vi "UHR-Fleezers Control (host) - 10.0.vi"() -> ()   [LabVIEW 2009] (continued)
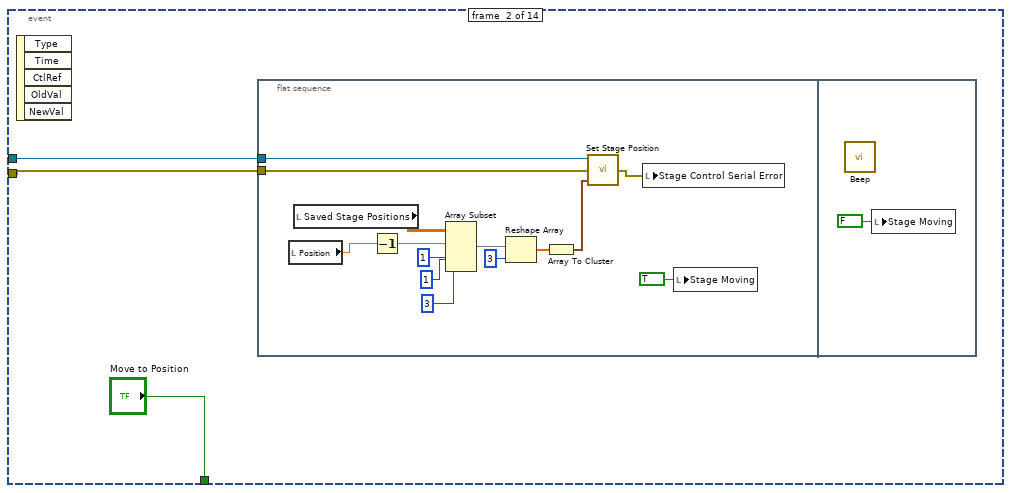
[diagram p2: hidden frame]
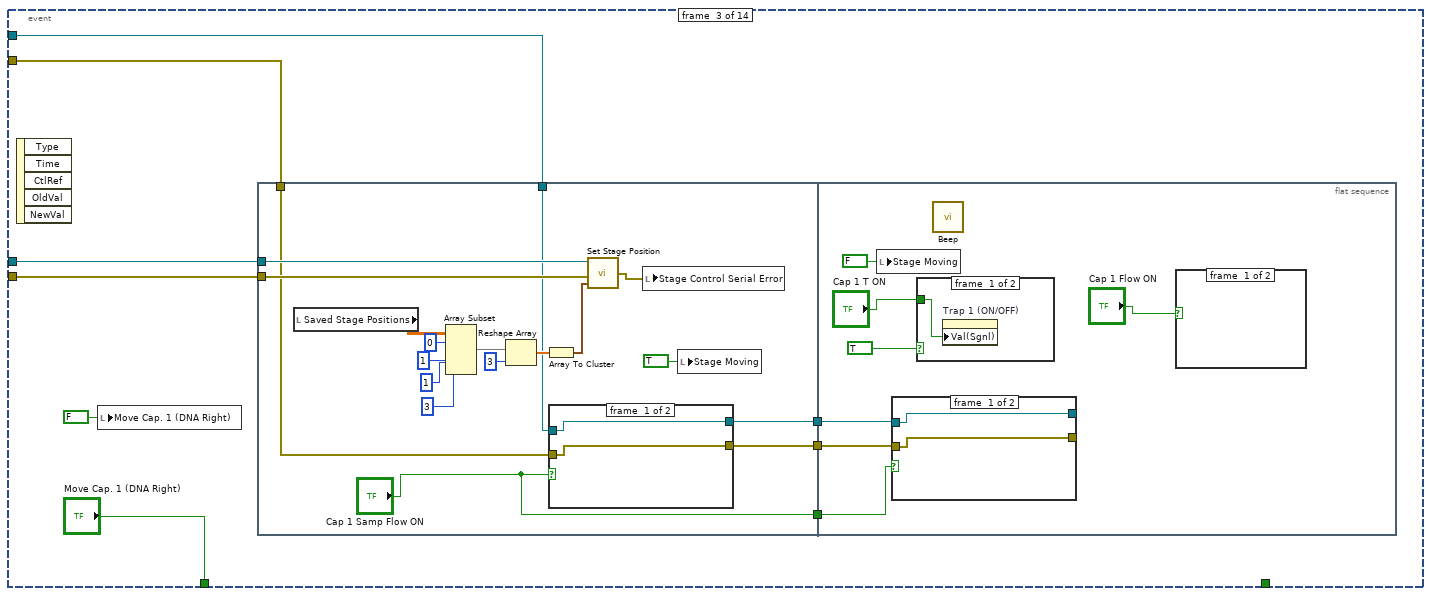
[diagram p3: hidden frame]
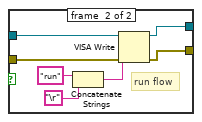
[diagram p4: hidden frame]
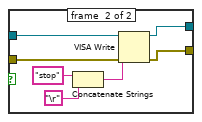
[diagram p5: hidden frame]
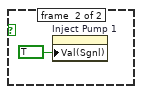
[diagram p6: hidden frame]
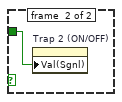
[diagram p7: hidden frame]
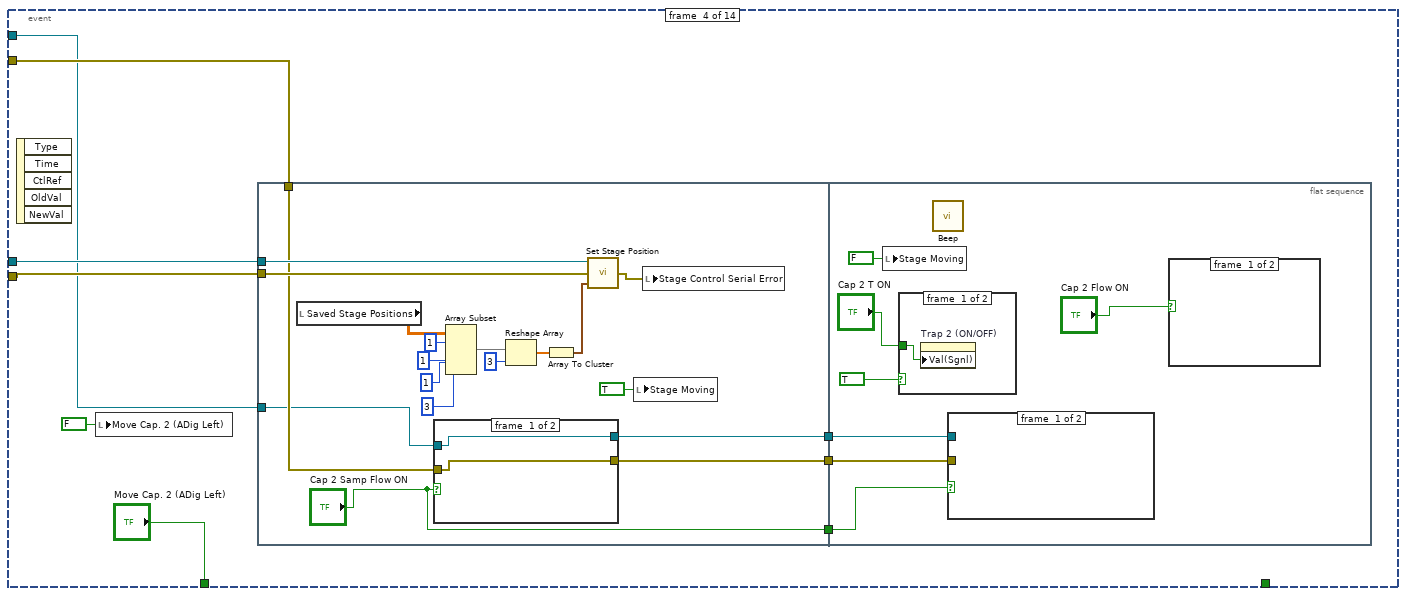
[diagram p8: hidden frame]
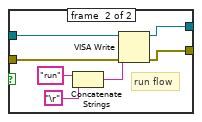
[diagram p9: hidden frame]
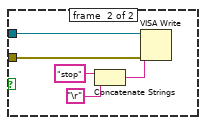
[diagram p10: hidden frame]
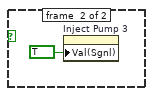
[diagram p11: hidden frame]
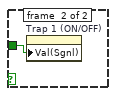
[diagram p12: hidden frame]
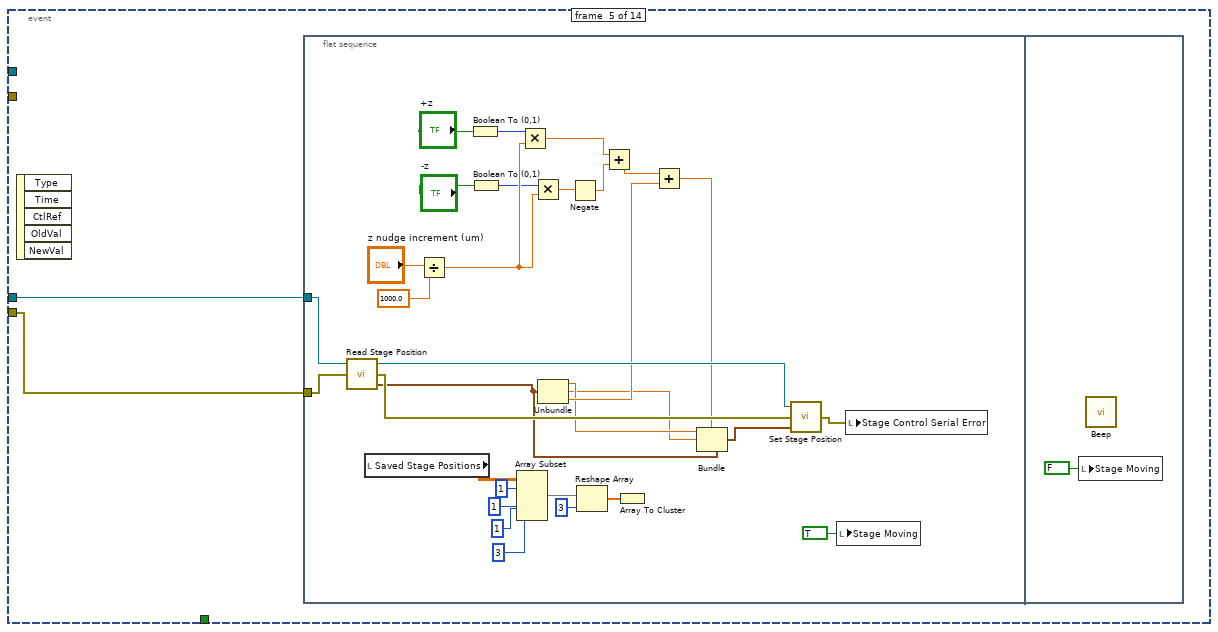
[diagram p13: hidden frame]
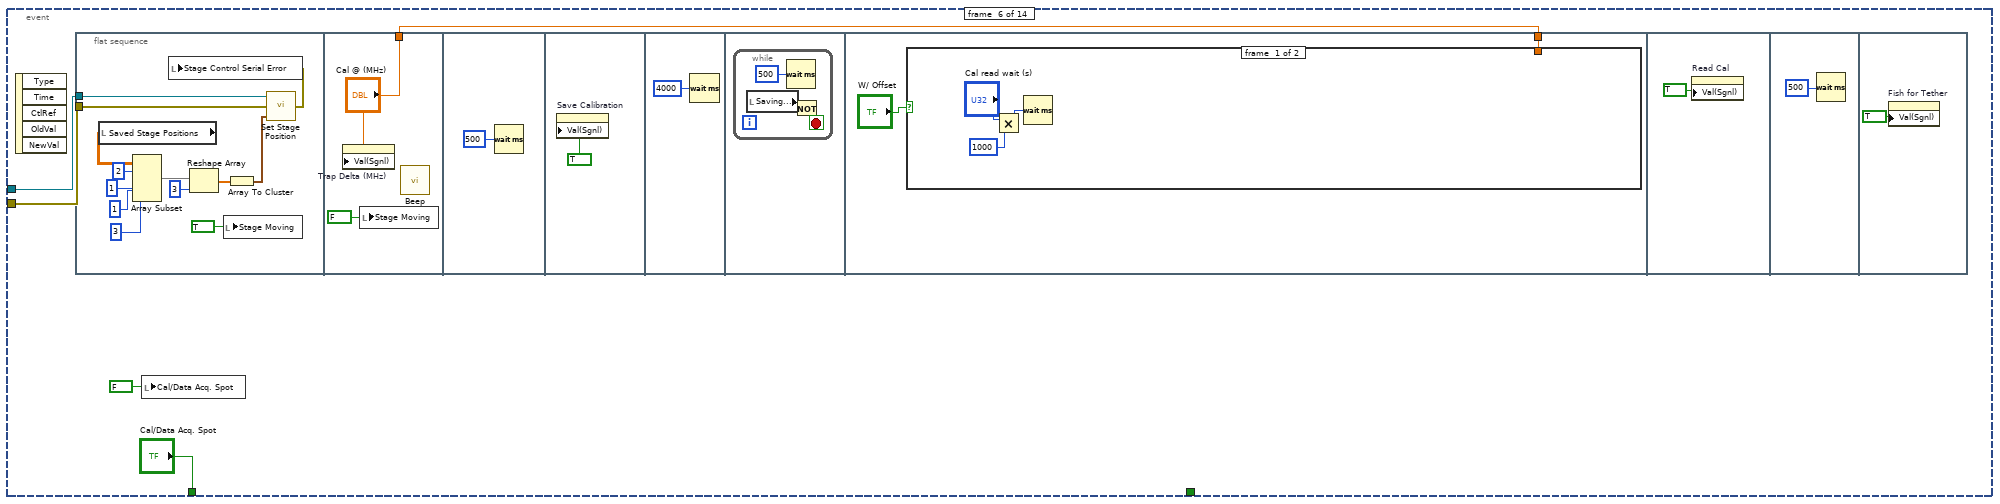
[diagram p14: hidden frame]
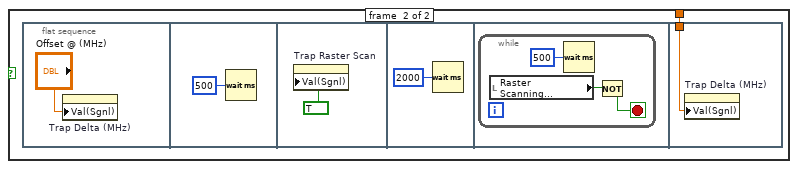
[diagram p15: hidden frame]
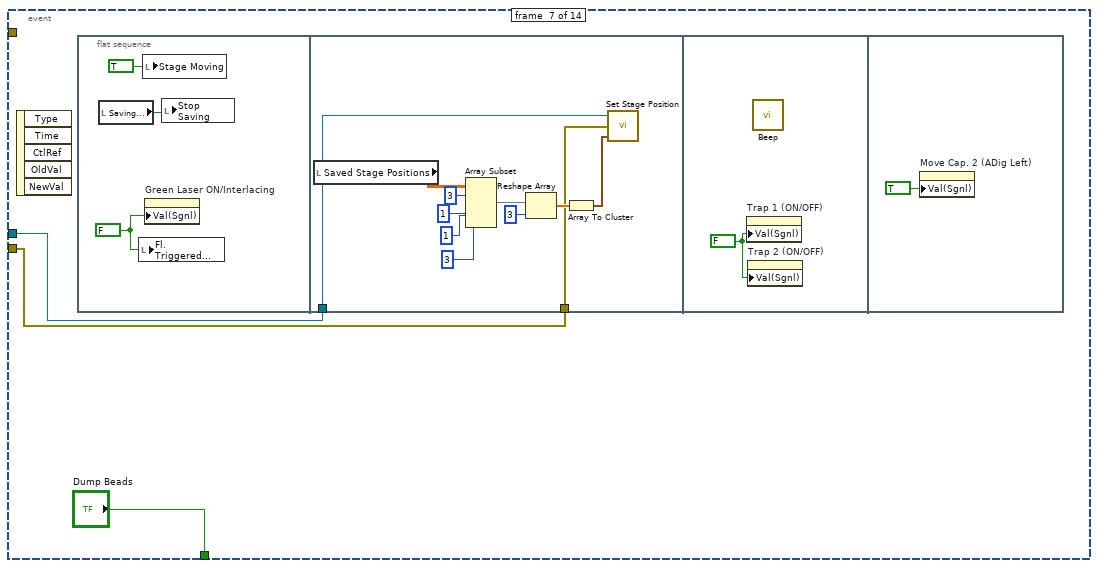
[diagram p16: hidden frame]
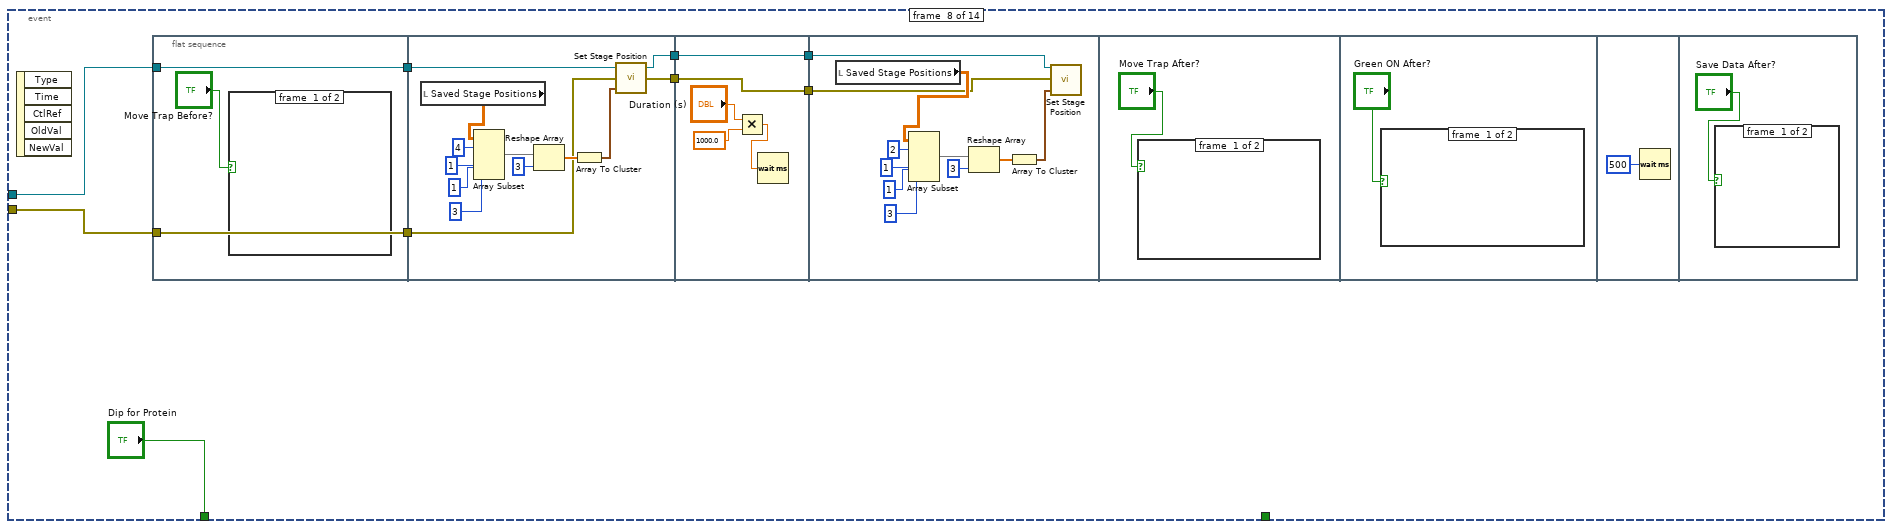
[diagram p17: hidden frame]
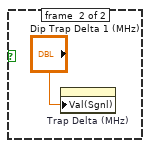
[diagram p18: hidden frame]
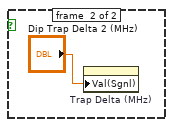
[diagram p19: hidden frame]
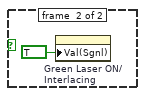
[diagram p20: hidden frame]
                          n1924 = local write "BD 2 Frequency 1 (MHz)"(w8168) -> ()
                          n1925 = local write "BD 1 Frequency 1 (MHz)"(w8170) -> ()
                        }
                      }
                    }
                    frame #1 {
                    }
                  }
                }
                event #1 {
                  n1926 = event-data() -> ("Button"=w8173:u16)  [unwired: 8 out]
                  n1927 = case shown="3" w8173 {
                    tunnel: [FALSE TRUE] -> w8174
                    frame #0 {
                    }
                    frame #1 {
                      n1928 = local write "Manipulating Trap"(FALSE ("Manipulating Trap")) -> ()
                    }
                  }
                }
              }
            }
          }
        }
      }
      event #1 {
        n1929 = event-data() -> ()  [unwired: 6 out]
      }
    }
    n1930 = local read "Stop All"() -> (w7995:bool)
    n1931 = node-c288() -> ()  [unwired: 2 out]
  }
  n1932 = timed-loop "Run Scripts, including: stage motion" {
    tunnel: w44 -> [w8180]
    tunnel: w43 -> [w8181]
    tunnel: [w8181] -> w42
    tunnel: [w8180] -> w41
    timing: w39 -> [_]
    timing-out: [_] -> w38
    tunnel: w22 -> [w8179]
    tunnel: w23 -> [w8178]
    stop <- w8182 stop-if-true
    n1933 = node-c288() -> ()  [unwired: 1 in, 1 out]
    n1934 = event shown="[10] \"Got ADig bead\": Value Change" {
      selector: _ -> [_ _ _ _ _ _ _ _ _ _ _ _ _ _]
      dyn-events: _ -> [_ _ _ _ _ _ _ _ _ _ _ _ _ _]
      timeout: _ -> [_ _ _ _ _ _ _ _ _ _ _ _ _ _]
      tunnel: ["Set Position" "Move to Position" "Move Cap. 1 (DNA Right)" "Move Cap. 2 (ADig Left)" _ "Cal/Data Acq. Spot" "Dump Beads" "Dip for Protein" _ _ "Got ADig bead" "Got DNA bead" "Take Detection Laser\nImage" _] -> _
      tunnel: [_ _ _ _ _ _ _ _ _ _ _ _ _ w8600] -> w8182
      tunnel: w8180 -> [w8200 w8208 w8232 w8287 w8332 w8368 w8409 w8434 w8484 w8510 _ _ _ _]
      tunnel: w8181 -> [w8201 w8209 w8233 w8288 w8333 w8369 w8410 w8435 w8485 w8511 _ _ _ _]
      tunnel: w8179 -> [_ _ w8230 w8284 _ _ _ _ _ _ _ _ _ _]
      tunnel: w8178 -> [_ _ w8229 w8285 _ _ _ _ _ _ _ _ _ _]
      event #0 {
        n1935 = event-data() -> ()  [unwired: 1 in, 5 out]
        n1936 = Build Array("Set Position 1", "Set Position 2", "Set Position 3", "Set Position 4", "Set Position 5") -> (w8199:bool[])
        n1937 = Boolean Array To Number(Boolean array=w8199) -> (number=w8198:u32)
        n1938 = Logarithm Base 2(1:w8198) -> (0:w8190:dbl)
        n1939 = call "Read Stage Position.vi"("error in"=w8200, "VISA resource name in"=w8201) -> ("Current Position"=w8205:cluster{dbl, dbl, dbl}, "error out"=w8204:errorcluster)  [unwired: 2 out]
        n1940 = Decrement(x="Position") -> (x-1=w8188:dbl)
        n1941 = Greater Or Equal?(x=w8190, y=0.0) -> (x >= y?=w8191:bool)
        n1942 = local write "Stage Control Serial Error"(w8204) -> ()
        n1943 = Cluster To Array(cluster=w8205) -> (array=w8202:dbl[])
        n1944 = Select(t=w8190, s=w8191, f=w8188) -> (s? t:f=w8187:dbl)
        n1945 = Increment(x=w8187) -> (x+1=w8186:dbl)
        n1946 = Build Array (concatenate)(w8186, w8202) -> (w8185:dbl[])
        n1947 = Replace Array Subset(array="Saved Stage Positions", new element=w8185, index (row)=w8187) -> (w8203:dbl[][])  [unwired: 1 in]
        n1948 = local write "Saved Stage Positions"(w8203) -> ()
      }
      event #1 {
        n1949 = event-data() -> ()  [unwired: 1 in, 5 out]
        n1950 = flat-sequence {
          tunnel: w8209 -> [w8212]
          tunnel: w8208 -> [w8211]
          frame #0 {
            n1951 = local read "Position"() -> (w8224:dbl)
            n1952 = local read "Saved Stage Positions"() -> (w8222:dbl[][])
            n1953 = Decrement(x=w8224) -> (x-1=w8221:dbl)
            n1954 = Array Subset(array=w8222, index (row)=w8221, length (row)=1 ("length"), index (col)=1 ("index"), length (col)=3 ("length")) -> (w8218:dbl[][])
            n1955 = Reshape Array(w8218, 3 ("dimension size")) -> (w8216:dbl[])
            n1956 = Array To Cluster(array=w8216) -> (cluster=w8215:cluster{"[0]":dbl, "[1]":dbl, "[2]":dbl})
            n1957 = call "Set Stage Position.vi"("Position"=w8215, "error in"=w8211, "VISA resource name in"=w8212) -> ("error out"=w8214:errorcluster)  [unwired: 2 out]
            n1958 = local write "Stage Control Serial Error"(w8214) -> ()
            n1959 = local write "Stage Moving"(TRUE ("Stage Moving")) -> ()
          }
          frame #1 {
            n1960 = call <vilib>:"Beep.vi"() -> ()  [unwired: 3 in, 9 out]
            n1961 = local write "Stage Moving"(FALSE ("Stage Moving")) -> ()
          }
        }
      }
      event #2 {
        n1962 = event-data() -> ()  [unwired: 1 in, 5 out]
        n1963 = local write "Move Cap. 1 (DNA Right)"(FALSE ("Move Cap. 1 (DNA Right)")) -> ()
        n1964 = flat-sequence {
          tunnel: w8233 -> [w8241]
          tunnel: w8232 -> [w8240]
          tunnel: w8230 -> [w8239]
          tunnel: w8229 -> [w8238]
          tunnel: [w8237] -> w8228
          tunnel: [w8236] -> w8227
          tunnel: ["Cap 1 Samp Flow ON"] -> w8226
          tunnel: w8228 -> [w8264]
          tunnel: w8227 -> [w8263]
          tunnel: w8226 -> [w8262]
          frame #0 {
            n1965 = local read "Saved Stage Positions"() -> (w8251:dbl[][])
            n1966 = Array Subset(array=w8251, index (row)=0 ("index"), length (row)=1 ("length"), index (col)=1 ("index"), length (col)=3 ("length")) -> (w8248:dbl[][])
            n1967 = Reshape Array(w8248, 3 ("dimension size")) -> (w8246:dbl[])
            n1968 = Array To Cluster(array=w8246) -> (cluster=w8245:cluster{"[0]":dbl, "[1]":dbl, "[2]":dbl})
            n1969 = case shown="True" "Cap 1 Samp Flow ON" {
              tunnel: w8238 -> [w8253 w8259]
              tunnel: w8239 -> [w8254 w8258]
              tunnel: [w8254 w8256] -> w8237
              tunnel: [w8253 w8255] -> w8236
              frame #0 {
              }
              frame #1 {
                # "run flow"
                n1970 = Concatenate Strings("run" ("string"), "\r") -> (w8260:string)
                n1971 = VISA Write(VISA resource name=w8258, write buffer=w8260, error in (no error)=w8259) -> (VISA resource name out=w8256:refnum<visa-resource-name>, error out=w8255:errorcluster)  [unwired: 1 out]
              }
            }
            n1972 = call "Set Stage Position.vi"("Position"=w8245, "error in"=w8240, "VISA resource name in"=w8241) -> ("error out"=w8244:errorcluster)  [unwired: 2 out]
            n1973 = local write "Stage Control Serial Error"(w8244) -> ()
            n1974 = local write "Stage Moving"(TRUE ("Stage Moving")) -> ()
          }
          frame #1 {
            n1975 = local write "Stage Moving"(FALSE ("Stage Moving")) -> ()
            n1976 = case shown="True" w8262 {
              tunnel: w8263 -> [w8269 w8275]
              tunnel: w8264 -> [w8270 w8274]
              tunnel: [w8270 w8272] -> _
              tunnel: [w8269 w8271] -> _
              frame #0 {
              }
              frame #1 {
                n1977 = Concatenate Strings("stop" ("string"), "\r") -> (w8276:string)
                n1978 = VISA Write(VISA resource name=w8274, write buffer=w8276, error in (no error)=w8275) -> (VISA resource name out=w8272:refnum<visa-resource-name>, error out=w8271:errorcluster)  [unwired: 1 out]
              }
            }
            n1979 = case shown="True" TRUE {
              tunnel: "Cap 1 T ON" -> [w8279 w8280]
              frame #0 {
                n1980 = property on="Trap 1 (ON/OFF)" class="Bool (strict)"("Val(Sgnl)"=w8279) -> ()  [unwired: 2 in, 2 out]
              }
              frame #1 {
                n1981 = property on="Trap 2 (ON/OFF)" class="Bool (strict)"("Val(Sgnl)"=w8280) -> ()  [unwired: 2 in, 2 out]
              }
            }
            n1982 = call <vilib>:"Beep.vi"() -> ()  [unwired: 3 in, 9 out]
            n1983 = case shown="True" "Cap 1 Flow ON" {
              frame #0 {
              }
              frame #1 {
                n1984 = property on="Inject Pump 1" class="Bool (strict)"("Val(Sgnl)"=TRUE ("Value (Signaling)")) -> ()  [unwired: 2 in, 2 out]
              }
            }
          }
        }
      }
      event #3 {
        n1985 = event-data() -> ()  [unwired: 1 in, 5 out]
        n1986 = local write "Move Cap. 2 (ADig Left)"(FALSE ("Move Cap. 2 (ADig Left)")) -> ()
        n1987 = flat-sequence {
          tunnel: w8288 -> [w8296]
          tunnel: w8287 -> [w8295]
          tunnel: w8285 -> [w8294]
          tunnel: w8284 -> [w8293]
          tunnel: [w8292] -> w8283
          tunnel: [w8291] -> w8282
          tunnel: ["Cap 2 Samp Flow ON"] -> w8281
          tunnel: w8283 -> [w8319]
          tunnel: w8282 -> [w8318]
          tunnel: w8281 -> [w8317]
          frame #0 {
            n1988 = local read "Saved Stage Positions"() -> (w8306:dbl[][])
            n1989 = case shown="True" "Cap 2 Samp Flow ON" {
              tunnel: w8294 -> [w8308 w8314]
              tunnel: w8293 -> [w8309 w8313]
              tunnel: [w8309 w8311] -> w8292
              tunnel: [w8308 w8310] -> w8291
              frame #0 {
              }
              frame #1 {
                # "run flow"
                n1990 = Concatenate Strings("run" ("string"), "\r") -> (w8315:string)
                n1991 = VISA Write(VISA resource name=w8313, write buffer=w8315, error in (no error)=w8314) -> (VISA resource name out=w8311:refnum<visa-resource-name>, error out=w8310:errorcluster)  [unwired: 1 out]
              }
            }
            n1992 = Array Subset(array=w8306, index (row)=1 ("index"), length (row)=1 ("length"), index (col)=1 ("index"), length (col)=3 ("length")) -> (w8303:dbl[][])
            n1993 = Reshape Array(w8303, 3 ("dimension size")) -> (w8301:dbl[])
            n1994 = Array To Cluster(array=w8301) -> (cluster=w8300:cluster{"[0]":dbl, "[1]":dbl, "[2]":dbl})
            n1995 = call "Set Stage Position.vi"("Position"=w8300, "error in"=w8295, "VISA resource name in"=w8296) -> ("error out"=w8299:errorcluster)  [unwired: 2 out]
            n1996 = local write "Stage Moving"(TRUE ("Stage Moving")) -> ()
            n1997 = local write "Stage Control Serial Error"(w8299) -> ()
          }
          frame #1 {
            n1998 = local write "Stage Moving"(FALSE ("Stage Moving")) -> ()
            n1999 = case shown="True" TRUE {
              tunnel: "Cap 2 T ON" -> [w8330 w8331]
              frame #0 {
                n2000 = property on="Trap 2 (ON/OFF)" class="Bool (strict)"("Val(Sgnl)"=w8330) -> ()  [unwired: 2 in, 2 out]
              }
              frame #1 {
                n2001 = property on="Trap 1 (ON/OFF)" class="Bool (strict)"("Val(Sgnl)"=w8331) -> ()  [unwired: 2 in, 2 out]
              }
            }
            n2002 = call <vilib>:"Beep.vi"() -> ()  [unwired: 3 in, 9 out]
            n2003 = case shown="True" w8317 {
              tunnel: w8319 -> [_ w8325]
              tunnel: w8318 -> [_ w8324]
              frame #0 {
              }
              frame #1 {
                n2004 = Concatenate Strings("stop" ("string"), "\r") -> (w8327:string)
                n2005 = VISA Write(VISA resource name=w8325, write buffer=w8327, error in (no error)=w8324) -> ()  [unwired: 3 out]
              }
            }
            n2006 = case shown="True" "Cap 2 Flow ON" {
              frame #0 {
              }
              frame #1 {
                n2007 = property on="Inject Pump 3" class="Bool (strict)"("Val(Sgnl)"=TRUE ("Value (Signaling)")) -> ()  [unwired: 2 in, 2 out]
              }
            }
          }
        }
      }
      event #4 {
        n2008 = event-data() -> ()  [unwired: 1 in, 5 out]
        n2009 = flat-sequence {
          tunnel: w8332 -> [w8354]
          tunnel: w8333 -> [w8334]
          frame #0 {
            n2010 = call "Read Stage Position.vi"("error in"=w8354, "VISA resource name in"=w8334) -> ("Current Position"=w8339:cluster{dbl, dbl, dbl}, "error out"=w8352:errorcluster, "VISA resource name out"=w8353:refnum<visa-resource-name>)  [unwired: 1 out]
            n2011 = local read "Saved Stage Positions"() -> (w8363:dbl[][])
            n2012 = Divide(x="z nudge increment (um)", y=1000.0) -> (x/y=w8351:dbl)
            n2013 = Boolean To (0,1)(Boolean="+z") -> (0, 1=w8343:i16)
            n2014 = Boolean To (0,1)(Boolean="-z") -> (0, 1=w8344:i16)
            n2015 = Array Subset(array=w8363, index (row)=1 ("index"), length (row)=1 ("length"), index (col)=1 ("index"), length (col)=3 ("length")) -> (w8360:dbl[][])
            n2016 = Multiply(x=w8343, y=w8351) -> (x*y=w8347:dbl)
            n2017 = Multiply(x=w8344, y=w8351) -> (x*y=w8345:dbl)
            n2018 = Unbundle(w8339) -> (w8337:dbl, w8336:dbl, w8340:dbl)
            n2019 = Negate(x=w8345) -> (-x=w8346:dbl)
            n2020 = Reshape Array(w8360, 3 ("dimension size")) -> (w8358:dbl[])
            n2021 = Add(x=w8347, y=w8346) -> (x+y=w8348:dbl)
            n2022 = Array To Cluster(array=w8358) -> ()  [unwired: 1 out]
            n2023 = Add(x=w8348, y=w8340) -> (x+y=w8338:dbl)
            n2024 = Bundle(cluster=w8339, w8337, w8336, w8338) -> (w8335:cluster{dbl, dbl, dbl})
            n2025 = call "Set Stage Position.vi"("Position"=w8335, "error in"=w8352, "VISA resource name in"=w8353) -> ("error out"=w8357:errorcluster)  [unwired: 2 out]
            n2026 = local write "Stage Moving"(TRUE ("Stage Moving")) -> ()
            n2027 = local write "Stage Control Serial Error"(w8357) -> ()
          }
          frame #1 {
            n2028 = local write "Stage Moving"(FALSE ("Stage Moving")) -> ()
            n2029 = call <vilib>:"Beep.vi"() -> ()  [unwired: 3 in, 9 out]
          }
        }
      }
      event #5 {
        n2030 = event-data() -> ()  [unwired: 1 in, 5 out]
        n2031 = flat-sequence {
          tunnel: w8369 -> [w8372]
          tunnel: w8368 -> [w8371]
          tunnel: ["Cal @ (MHz)"] -> w8367
          tunnel: w8367 -> [w8392]
          frame #0 {
            n2032 = local read "Saved Stage Positions"() -> (w8375:dbl[][])
            n2033 = Array Subset(array=w8375, index (row)=2 ("index"), length (row)=1 ("length"), index (col)=1 ("index"), length (col)=3 ("length")) -> (w8378:dbl[][])
            n2034 = Reshape Array(w8378, 3 ("dimension size")) -> (w8380:dbl[])
            n2035 = local write "Stage Moving"(TRUE ("Stage Moving")) -> ()
            n2036 = Array To Cluster(array=w8380) -> (cluster=w8381:cluster{"[0]":dbl, "[1]":dbl, "[2]":dbl})
            n2037 = call "Set Stage Position.vi"("Position"=w8381, "error in"=w8371, "VISA resource name in"=w8372) -> ("error out"=w8382:errorcluster)  [unwired: 2 out]
            n2038 = local write "Stage Control Serial Error"(w8382) -> ()
          }
          frame #1 {
            n2039 = property on="Trap Delta (MHz)" class="DigNum (strict)"("Val(Sgnl)"="Cal @ (MHz)") -> ()  [unwired: 2 in, 2 out]
            n2040 = local write "Stage Moving"(FALSE ("Stage Moving")) -> ()
            n2041 = call <vilib>:"Beep.vi"() -> ()  [unwired: 3 in, 9 out]
          }
          frame #2 {
            n2042 = Wait (ms)(milliseconds to wait=u32 500) -> ()  [unwired: 1 out]
          }
          frame #3 {
            n2043 = property on="Save Calibration" class="Bool (strict)"("Val(Sgnl)"=TRUE ("Value (Signaling)")) -> ()  [unwired: 2 in, 2 out]
          }
          frame #4 {
            n2044 = Wait (ms)(milliseconds to wait=u32 4000) -> ()  [unwired: 1 out]
          }
          frame #5 {
            n2045 = while {
              stop <- w8389 stop-if-true
              n2046 = local read "Saving..."() -> (w8390:bool)
              n2047 = Wait (ms)(milliseconds to wait=u32 500) -> ()  [unwired: 1 out]
              n2048 = Not(x=w8390) -> (.not. x?=w8389:bool)
            }
          }
          frame #6 {
            n2049 = case shown="True" "W/ Offset" {
              tunnel: w8392 -> [_ w8397]
              frame #0 {
                n2050 = Multiply(x="Cal read wait (s)", y=u32 1000 ("milliseconds to wait")) -> (x*y=w8395:u32)
                n2051 = Wait (ms)(milliseconds to wait=w8395) -> ()  [unwired: 1 out]
              }
              frame #1 {
                n2052 = flat-sequence {
                  tunnel: w8397 -> [w8405]
                  frame #0 {
                    n2053 = property on="Trap Delta (MHz)" class="DigNum (strict)"("Val(Sgnl)"="Offset @ (MHz)") -> ()  [unwired: 2 in, 2 out]
                  }
                  frame #1 {
                    n2054 = Wait (ms)(milliseconds to wait=u32 500) -> ()  [unwired: 1 out]
                  }
                  frame #2 {
                    n2055 = property on="Trap Raster Scan" class="Bool (strict)"("Val(Sgnl)"=TRUE ("Value (Signaling)")) -> ()  [unwired: 2 in, 2 out]
                  }
                  frame #3 {
                    n2056 = Wait (ms)(milliseconds to wait=u32 2000) -> ()  [unwired: 1 out]
                  }
                  frame #4 {
                    n2057 = while {
                      stop <- w8403 stop-if-true
                      n2058 = local read "Raster Scanning..."() -> (w8404:bool)
                      n2059 = Wait (ms)(milliseconds to wait=u32 500) -> ()  [unwired: 1 out]
                      n2060 = Not(x=w8404) -> (.not. x?=w8403:bool)
                    }
                  }
                  frame #5 {
                    n2061 = property on="Trap Delta (MHz)" class="DigNum (strict)"("Val(Sgnl)"=w8405) -> ()  [unwired: 2 in, 2 out]
                  }
                }
              }
            }
          }
          frame #7 {
            n2062 = property on="Read Cal" class="Bool (strict)"("Val(Sgnl)"=TRUE ("Value (Signaling)")) -> ()  [unwired: 2 in, 2 out]
          }
          frame #8 {
            n2063 = Wait (ms)(milliseconds to wait=u32 500) -> ()  [unwired: 1 out]
          }
          frame #9 {
            n2064 = property on="Fish for Tether" class="Bool (strict)"("Val(Sgnl)"=TRUE ("Value (Signaling)")) -> ()  [unwired: 2 in, 2 out]
          }
        }
        n2065 = local write "Cal/Data Acq. Spot"(FALSE ("Cal/Data Acq. Spot")) -> ()
      }
      event #6 {
        n2066 = event-data() -> ()  [unwired: 1 in, 5 out]
        n2067 = flat-sequence {
          tunnel: w8410 -> [w8416]
          tunnel: w8409 -> [w8415]
          frame #0 {
            w8412 = FALSE ("Fl. Triggered...")
            n2068 = local read "Saving..."() -> (w8413:bool)
            n2069 = local write "Fl. Triggered..."(w8412) -> ()
            n2070 = local write "Stage Moving"(TRUE ("Stage Moving")) -> ()
            n2071 = property on="Green Laser ON/Interlacing" class="Bool (strict)"("Val(Sgnl)"=w8412) -> ()  [unwired: 2 in, 2 out]
            n2072 = local write "Stop Saving"(w8413) -> ()
          }
          frame #1 {
            n2073 = local read "Saved Stage Positions"() -> (w8417:dbl[][])
            n2074 = Array Subset(array=w8417, index (row)=3 ("index"), length (row)=1 ("length"), index (col)=1 ("index"), length (col)=3 ("length")) -> (w8422:dbl[][])
            n2075 = Reshape Array(w8422, 3 ("dimension size")) -> (w8420:dbl[])
            n2076 = Array To Cluster(array=w8420) -> (cluster=w8419:cluster{"[0]":dbl, "[1]":dbl, "[2]":dbl})
            n2077 = call "Set Stage Position.vi"("Position"=w8419, "error in"=w8415, "VISA resource name in"=w8416) -> ()  [unwired: 3 out]
          }
          frame #2 {
            w8426 = FALSE ("Value (Signaling)")
            n2078 = property on="Trap 1 (ON/OFF)" class="Bool (strict)"("Val(Sgnl)"=w8426) -> ()  [unwired: 2 in, 2 out]
            n2079 = property on="Trap 2 (ON/OFF)" class="Bool (strict)"("Val(Sgnl)"=w8426) -> ()  [unwired: 2 in, 2 out]
            n2080 = call <vilib>:"Beep.vi"() -> ()  [unwired: 3 in, 9 out]
          }
          frame #3 {
            n2081 = property on="Move Cap. 2 (ADig Left)" class="Bool (strict)"("Val(Sgnl)"=TRUE ("Value (Signaling)")) -> ()  [unwired: 2 in, 2 out]
          }
        }
      }
      event #7 {
        n2082 = event-data() -> ()  [unwired: 1 in, 5 out]
        n2083 = flat-sequence {
          tunnel: w8434 -> [w8438]
          tunnel: w8435 -> [w8439]
          tunnel: [w8439] -> w8429
          tunnel: [w8438] -> w8428
          tunnel: [w8442] -> w8432
          tunnel: [w8441] -> w8430
          tunnel: w8429 -> [w8445]
          tunnel: w8428 -> [w8444]
          tunnel: [w8455] -> w8433
          tunnel: w8432 -> [w8455]
          tunnel: [w8454] -> w8431
          tunnel: w8430 -> [w8454]
          tunnel: w8433 -> [w8460]
          tunnel: w8431 -> [w8459]
          frame #0 {
            n2084 = case shown="True" "Move Trap Before?" {
              frame #0 {
              }
              frame #1 {
                n2085 = property on="Trap Delta (MHz)" class="DigNum (strict)"("Val(Sgnl)"="Dip Trap Delta 1 (MHz)") -> ()  [unwired: 2 in, 2 out]
              }
            }
          }
          frame #1 {
            n2086 = local read "Saved Stage Positions"() -> (w8443:dbl[][])
            n2087 = Array Subset(array=w8443, index (row)=4 ("index"), length (row)=1 ("length"), index (col)=1 ("index"), length (col)=3 ("length")) -> (w8450:dbl[][])
            n2088 = Reshape Array(w8450, 3 ("dimension size")) -> (w8448:dbl[])
            n2089 = Array To Cluster(array=w8448) -> (cluster=w8447:cluster{"[0]":dbl, "[1]":dbl, "[2]":dbl})
            n2090 = call "Set Stage Position.vi"("Position"=w8447, "error in"=w8444, "VISA resource name in"=w8445) -> ("error out"=w8441:errorcluster, "VISA resource name out"=w8442:refnum<visa-resource-name>)  [unwired: 1 out]
          }
          frame #2 {
            n2091 = Multiply(x="Duration (s)", y=1000.0) -> (x*y=w8456:dbl)
            n2092 = Wait (ms)(milliseconds to wait=w8456) -> ()  [unwired: 1 out]
          }
          frame #3 {
            n2093 = local read "Saved Stage Positions"() -> (w8461:dbl[][])
            n2094 = Array Subset(array=w8461, index (row)=2 ("index"), length (row)=1 ("length"), index (col)=1 ("index"), length (col)=3 ("length")) -> (w8466:dbl[][])
            n2095 = Reshape Array(w8466, 3 ("dimension size")) -> (w8464:dbl[])
            n2096 = Array To Cluster(array=w8464) -> (cluster=w8463:cluster{"[0]":dbl, "[1]":dbl, "[2]":dbl})
            n2097 = call "Set Stage Position.vi"("Position"=w8463, "error in"=w8459, "VISA resource name in"=w8460) -> ()  [unwired: 3 out]
          }
          frame #4 {
            n2098 = case shown="True" "Move Trap After?" {
              frame #0 {
              }
              frame #1 {
                n2099 = property on="Trap Delta (MHz)" class="DigNum (strict)"("Val(Sgnl)"="Dip Trap Delta 2 (MHz)") -> ()  [unwired: 2 in, 2 out]
              }
            }
          }
          frame #5 {
            n2100 = case shown="True" "Green ON After?" {
              frame #0 {
              }
              frame #1 {
                n2101 = property on="Green Laser ON/Interlacing" class="Bool (strict)"("Val(Sgnl)"=TRUE ("Value (Signaling)")) -> ()  [unwired: 2 in, 2 out]
              }
            }
          }
          frame #6 {
            n2102 = Wait (ms)(milliseconds to wait=u32 500) -> ()  [unwired: 1 out]
          }
          frame #7 {
            n2103 = case shown="True" "Save Data After?" {
              frame #0 {
              }
              frame #1 {
                n2104 = property on="Start Saving" class="Bool (strict)"("Val(Sgnl)"=TRUE ("Value (Signaling)")) -> ()  [unwired: 2 in, 2 out]
              }
            }
          }
        }
      }
      event #8 {
        n2105 = event-data() -> ()  [unwired: 1 in, 5 out]
        n2106 = flat-sequence {
          tunnel: w8485 -> [w8488]
          tunnel: w8484 -> [w8496]
          tunnel: [w8490] -> w8483
          tunnel: [w8489] -> w8482
          tunnel: [w8487] -> w8480
          tunnel: [w8486] -> w8477
          tunnel: w8483 -> [w8503]
          tunnel: w8482 -> [w8502]
          tunnel: [w8500] -> w8481
          tunnel: w8480 -> [w8501]
          tunnel: [w8499] -> w8479
          tunnel: [w8498] -> w8478
          tunnel: w8477 -> [w8498]
          tunnel: w8481 -> [w8507]
          tunnel: w8479 -> [w8506]
          tunnel: w8478 -> [w8505]
          frame #0 {
            n2107 = call "Read Stage Position.vi"("error in"=w8496, "VISA resource name in"=w8488) -> ("Current Position"=w8486:cluster{dbl, dbl, dbl}, "error out"=w8489:errorcluster, "VISA resource name out"=w8487:refnum<visa-resource-name>)  [unwired: 1 out]
            "Current Position" <- w8486
            n2108 = local write "Stage Control Serial Error"(w8489) -> ()
            n2109 = Unbundle(w8486) -> (w8493:dbl, w8495:dbl, w8491:dbl)
            n2110 = Add(x=w8495, y="Y change (mm)") -> (x+y=w8492:dbl)
            n2111 = Bundle(w8493, w8492, w8491) -> (w8490:cluster{dbl, dbl, dbl})  [unwired: 1 in]
          }
          frame #1 {
            # "move to new position and start saving"
            n2112 = local write "Stage Moving"(TRUE ("Stage Moving")) -> ()
            n2113 = local write "Start Saving"(TRUE ("Start Saving")) -> ()
            n2114 = call "Set Stage Position.vi"("Position"=w8503, "error in"=w8502, "VISA resource name in"=w8501) -> ("error out"=w8499:errorcluster, "VISA resource name out"=w8500:refnum<visa-resource-name>)  [unwired: 1 out]
          }
          frame #2 {
            # "go back to start"
            n2115 = call "Set Stage Position.vi"("Position"=w8505, "error in"=w8506, "VISA resource name in"=w8507) -> ()  [unwired: 3 out]
          }
          frame #3 {
            # "stop saving"
            n2116 = local write "Stop Saving"(TRUE ("Stop Saving")) -> ()
            n2117 = local write "Stage Moving"(FALSE ("Stage Moving")) -> ()
          }
        }
      }
      event #9 {
        n2118 = event-data() -> ()  [unwired: 1 in, 5 out]
        n2119 = Or(x="Move to Position 5", y="Lower Ch. Cap.") -> (x .or. y?=w8513:bool)
        n2120 = Build Array("Move to Position 1", "Move to Position 2", "Move to Position 3", "Move to Position 4", w8513) -> (w8516:bool[])
        n2121 = Boolean Array To Number(Boolean array=w8516) -> (number=w8515:u32)
        n2122 = Logarithm Base 2(1:w8515) -> (0:w8514:dbl)
        n2123 = flat-sequence {
          tunnel: w8514 -> [w8525]
          tunnel: w8511 -> [w8523]
          tunnel: w8510 -> [w8522]
          frame #0 {
            n2124 = local read "Saved Stage Positions"() -> (w8533:dbl[][])
            n2125 = Array Subset(array=w8533, index (row)=w8525, length (row)=1 ("length"), index (col)=1 ("index"), length (col)=3 ("length")) -> (w8530:dbl[][])
            n2126 = Reshape Array(w8530, 3 ("dimension size")) -> (w8528:dbl[])
            n2127 = Array To Cluster(array=w8528) -> (cluster=w8527:cluster{"[0]":dbl, "[1]":dbl, "[2]":dbl})
            n2128 = call "Set Stage Position.vi"("Position"=w8527, "error in"=w8522, "VISA resource name in"=w8523) -> ("error out"=w8526:errorcluster)  [unwired: 2 out]
            n2129 = local write "Stage Moving"(TRUE ("Stage Moving")) -> ()
            n2130 = local write "Stage Control Serial Error"(w8526) -> ()
          }
          frame #1 {
            n2131 = call <vilib>:"Beep.vi"() -> ()  [unwired: 3 in, 9 out]
            n2132 = local write "Stage Moving"(FALSE ("Stage Moving")) -> ()
          }
        }
      }
      event #10 {
        n2133 = event-data() -> ()  [unwired: 1 in, 5 out]
        n2134 = property on="Move Cap. 1 (DNA Right)" class="Bool (strict)"("Val(Sgnl)"=TRUE ("Value (Signaling)")) -> ()  [unwired: 2 in, 2 out]
        n2135 = property on="Inject Pump 3" class="Bool (strict)"("Val(Sgnl)"=FALSE ("Value (Signaling)")) -> ()  [unwired: 2 in, 2 out]
      }
      event #11 {
        n2136 = event-data() -> ()  [unwired: 1 in, 5 out]
        n2137 = property on="Cal/Data Acq. Spot" class="Bool (strict)"("Val(Sgnl)"=TRUE ("Value (Signaling)")) -> ()  [unwired: 2 in, 2 out]
        n2138 = property on="Inject Pump 1" class="Bool (strict)"("Val(Sgnl)"=FALSE ("Value (Signaling)")) -> ()  [unwired: 2 in, 2 out]
      }
      event #12 {
        n2139 = event-data() -> ()  [unwired: 1 in, 5 out]
        n2140 = flat-sequence {
          tunnel: [w8567] -> w8557
          tunnel: [w8566] -> w8550
          tunnel: [w8565] -> w8542
          tunnel: [w8570] -> w8558
          tunnel: w8557 -> [w8570]
          tunnel: [w8569] -> w8551
          tunnel: w8550 -> [w8569]
          tunnel: [w8568] -> w8543
          tunnel: w8542 -> [w8568]
          tunnel: [w8574] -> w8559
          tunnel: w8558 -> [w8574]
          tunnel: [w8573] -> w8552
          tunnel: w8551 -> [w8573]
          tunnel: [w8572] -> w8544
          tunnel: w8543 -> [w8572]
          tunnel: [w8580] -> w8560
          tunnel: w8559 -> [w8580]
          tunnel: [w8579] -> w8553
          tunnel: w8552 -> [w8579]
          tunnel: [w8578] -> w8545
          tunnel: w8544 -> [w8578]
          tunnel: [w8584] -> w8561
          tunnel: w8560 -> [w8584]
          tunnel: [w8583] -> w8554
          tunnel: w8553 -> [w8583]
          tunnel: [w8582] -> w8546
          tunnel: w8545 -> [w8582]
          tunnel: [w8588] -> w8562
          tunnel: w8561 -> [w8588]
          tunnel: [w8587] -> w8555
          tunnel: w8554 -> [w8587]
          tunnel: [w8586] -> w8547
          tunnel: w8546 -> [w8586]
          tunnel: [w8592] -> w8563
          tunnel: w8562 -> [w8592]
          tunnel: [w8591] -> w8556
          tunnel: w8555 -> [w8591]
          tunnel: [w8590] -> w8548
          tunnel: w8547 -> [w8590]
          tunnel: w8563 -> [w8598]
          tunnel: w8556 -> [w8597]
          tunnel: [w8595] -> w8549
          tunnel: w8548 -> [w8595]
          tunnel: w8549 -> [w8599]
          frame #0 {
            n2141 = local read "Green Laser ON/Interlacing"() -> (w8567:bool)
            n2142 = local read "Green laser mode"() -> (w8566:enum32{"Laser ON", "Laser OFF", "Interlace"})
            n2143 = local read "Green FB On/Off"() -> (w8565:bool)
          }
          frame #1 {
            n2144 = property on="Green FB On/Off" class="Bool (strict)"("Val(Sgnl)"=FALSE ("Value (Signaling)")) -> ()  [unwired: 2 in, 2 out]
          }
          frame #2 {
            n2145 = property on="Green Laser ON/Interlacing" class="Bool (strict)"("Val(Sgnl)"=TRUE ("Value (Signaling)")) -> ()  [unwired: 2 in, 2 out]
            n2146 = property on="Flip Green Filter" class="Bool (strict)"("Val(Sgnl)"=TRUE ("Value (Signaling)")) -> ()  [unwired: 2 in, 2 out]
            n2147 = property on="Green laser mode" class="RadioBtnsControl (strict)"("Val(Sgnl)"=enum32{"Laser ON", "Laser OFF", "Interlace"}."Laser ON" ("Value (Signaling)")) -> ()  [unwired: 2 in, 2 out]
          }
          frame #3 {
            n2148 = Wait (ms)(milliseconds to wait=u32 500) -> ()  [unwired: 1 out]
          }
          frame #4 {
            n2149 = property on="Confocal Image" class="Bool (strict)"("Val(Sgnl)"=TRUE ("Value (Signaling)")) -> ()  [unwired: 2 in, 2 out]
          }
          frame #5 {
            n2150 = Wait (ms)(milliseconds to wait=u32 2000) -> ()  [unwired: 1 out]
          }
          frame #6 {
            n2151 = while {
              stop <- w8593 stop-if-true
              n2152 = local read "Saving..."() -> (w8594:bool)
              n2153 = Not(x=w8594) -> (.not. x?=w8593:bool)
            }
          }
          frame #7 {
            n2154 = property on="Flip Green Filter" class="Bool (strict)"("Val(Sgnl)"=TRUE ("Value (Signaling)")) -> ()  [unwired: 2 in, 2 out]
            n2155 = property on="Green Laser ON/Interlacing" class="Bool (strict)"("Val(Sgnl)"=w8598) -> ()  [unwired: 2 in, 2 out]
            n2156 = property on="Green laser mode" class="RadioBtnsControl (strict)"("Val(Sgnl)"=w8597) -> ()  [unwired: 2 in, 2 out]
          }
          frame #8 {
            n2157 = property on="Green FB On/Off" class="Bool (strict)"("Val(Sgnl)"=w8599) -> ()  [unwired: 2 in, 2 out]
          }
        }
      }
      event #13 {
        n2158 = event-data() -> ()  [unwired: 1 in, 5 out]
        n2159 = local read "Stop All"() -> (w8600:bool)
      }
    }
    n2160 = node-c288() -> ()  [unwired: 1 in, 1 out]
  }
  n2161 = node-c288(w51) -> ()  [unwired: 1 out]
  n2162 = node-c288(w53) -> ()  [unwired: 1 out]
  n2163 = node-c288(w38) -> ()  [unwired: 1 out]
  n2164 = VISA Close(VISA resource name=w42, error in (no error)=w41) -> (error out=w95:errorcluster)
  n2165 = call <vilib>:"Simple Error Handler.vi"("error in (no error)"=w95) -> ()  [unwired: 1 in, 8 out]
  n2166 = node-c288(w49) -> ()  [unwired: 1 out]
  n2167 = node-c288(w156) -> ()  [unwired: 1 out]
  n2168 = flat-sequence {
    tunnel: w252 -> [w8604]
    tunnel: w254 -> [w8605]
    tunnel: [w8603] -> w233
    tunnel: [w8602] -> w232
    tunnel: w213 -> [_]
    tunnel: w211 -> [_]
    tunnel: w164 -> [_]
    tunnel: w55 -> [_]
    tunnel: w233 -> [w8663]
    tunnel: w232 -> [w8664]
    frame #0 {
      w8601 = FALSE ("AI to FIFO")
      n2169 = xnode "Read/Write Control"("FPGA VI Reference In"=w8605, "error in"=w8604, "AI to FIFO"=w8601, "APD to FIFO"=w8601) -> ("FPGA VI Reference Out"=w8603:T20, "error out"=w8602:errorcluster)
    }
    frame #1 {
      n2170 = xnode "Close FPGA VI Reference"("FPGA VI Reference In"=w8663, "error in"=w8664) -> ("error out"=→"error out":errorcluster)
    }
  }
